vi "UHR-Fleezers Control (host) - 10.5.vi"() -> ()   [LabVIEW 2010] (continued)
        n1065 = local read "Scan Range (V)\n(of steps)"() -> (w2741:dbl)
        n1066 = property on="Scan Range (V)\n(of steps)" class="DigNum (strict)"("Val(Sgnl)"=w2741) -> ()  [unwired: 2 in, 2 out]
      }
    }
    n1067 = node-c288() -> ()  [unwired: 2 out]
  }
  n1068 = node-c288(3 ("Processor")) -> (w77:T25)  [unwired: 3 out]
  n1069 = disable-structure shown="Disabled" {
    disable-tunnel: [w4150 _] -> w13
    disable-tunnel: w9 -> [w4149 _]
    frame Disabled {
      n1070 = node-c288() -> (w4152:T25)  [unwired: 4 out]
      n1071 = timed-loop "Rough control of MCL mirror stage (debugging)" {
        tunnel: w4149 -> [w4155]
        tunnel: [w4154] -> w4150
        timing: w4152 -> [_]
        timing-out: [_] -> w4151
        stop <- w4154 stop-if-true
        n1072 = node-c288() -> ()  [unwired: 2 out]
        n1073 = case shown="1" "MCL Mode" {
          tunnel: w4155 -> [_ w4158 w4262]
          frame 0, Default {
          }
          frame 1 {
            n1074 = node-c288() -> (w4160:T25)  [unwired: 4 out]
            n1075 = timed-loop "Oscillate MCL mirror" {
              timing: w4160 -> [_]
              timing-out: [_] -> w4159
              tunnel: w4158 -> [w4199]
              i -> [w4198]
              stop <- w4161 stop-if-true
              n1076 = node-c288() -> (w4197:i64)  [unwired: 1 out]
              n1077 = Multiply(x="AO1", y=32767.0) -> (x*y=w4193:dbl)
              n1078 = Multiply(x="AO2", y=32767.0) -> (x*y=w4188:dbl)
              n1079 = Divide(x=w4193, y=10.0) -> (x/y=w4194:dbl)
              n1080 = Divide(x=w4188, y=10.0) -> (x/y=w4189:dbl)
              n1081 = To Word Integer(number=w4194) -> (16bit integer=w4186:i16)
              n1082 = To Word Integer(number=w4189) -> (16bit integer=w4185:i16)
              n1083 = Divide(x=w4197, y=i64 1000) -> (x/y=w4168:dbl)
              n1084 = Multiply(x=w4168, y=w4198) -> (x*y=w4179:dbl)
              n1085 = Multiply(x="Osc. freq. (Hz) 2", y=6.283185307179586) -> (x*y=w4180:dbl)
              n1086 = Multiply(x=w4180, y=w4179) -> (x*y=w4178:dbl)
              n1087 = Sine(x=w4178) -> (sin(x)=w4177:dbl)
              n1088 = Multiply(x=w4177, y="Osc. amp. (V)") -> (x*y=w4175:dbl)
              n1089 = Add(x=w4175, y="Osc. center (V)") -> (x+y=w4173:dbl)
              n1090 = Divide(x=w4173, y=10.0) -> (x/y=w4171:dbl)
              n1091 = Multiply(x=w4171, y=32767.0) -> (x*y=w4166:dbl)
              n1092 = Select(t=w4166, s="Scan axis", f=w4186) -> (s? t:f=w4184:dbl)
              n1093 = Select(t=w4185, s="Scan axis", f=w4166) -> (s? t:f=w4183:dbl)
              n1094 = local read "MCL Mode"() -> (w4165:u16)
              n1095 = Not Equal?(x=w4165, y=u16 1) -> (x != y?=w4162:bool)
              n1096 = local read "Stop All"() -> (w4163:bool)
              n1097 = xnode "Read/Write Control"("FPGA VI Reference In"=w4199, "AO1"=w4184, "AO2"=w4183) -> ()  [unwired: 1 in, 2 out]
              n1098 = Compound Arithmetic op=OR(w4163, w4162) -> (w4161:bool)
              n1099 = node-c288() -> ()  [unwired: 2 out]
            }
            n1100 = node-c288(w4159) -> ()  [unwired: 1 out]
          }
          frame 2 {
            n1101 = case shown="True" "Start Scan" {
              tunnel: w4262 -> [_ w4274]
              frame False {
              }
              frame True {
                n1102 = Subtract(x="End (V)", y="Begin (V)") -> (x-y=w4270:dbl)
                n1103 = Decrement(x="N Points") -> (x-1=w4269:dbl)
                n1104 = Divide(x=w4270, y=w4269) -> (x/y=w4267:dbl)
                n1105 = for {
                  N: "N Points" -> [_]
                  tunnel: "Begin (V)" -> [w4287]
                  tunnel: w4274 -> [w4279]
                  tunnel: [w4278] -> w4273 mode=indexing
                  tunnel: w4267 -> [w4277]
                  tunnel: [w4275] -> w4266 mode=indexing
                  i -> [w4286]
                  n1106 = Multiply(x=w4277, y=w4286) -> (x*y=w4285:dbl)
                  n1107 = Add(x=w4287, y=w4285) -> (x+y=w4282:dbl)
                  n1108 = local read "Scan axis"() -> (w4276:bool)
                  n1109 = local read "AO1"() -> (w4284:dbl)
                  n1110 = local read "AO2"() -> (w4283:dbl)
                  n1111 = Select(t=w4282, s=w4276, f=w4284) -> (s? t:f=w4281:dbl)
                  n1112 = Select(t=w4283, s=w4276, f=w4282) -> (s? t:f=w4280:dbl)
                  n1113 = flat-sequence {
                    tunnel: w4281 -> [w4291]
                    tunnel: w4280 -> [w4290]
                    tunnel: w4279 -> [w4288]
                    tunnel: [w4358] -> w4278
                    tunnel: [w4357] -> w4275
                    frame #0 {
                      w4294 = 10.0 ("y")
                      w4289 = 32767.0 ("y")
                      n1114 = Multiply(x=w4291, y=w4289) -> (x*y=w4297:dbl)
                      n1115 = Multiply(x=w4290, y=w4289) -> (x*y=w4295:dbl)
                      n1116 = Divide(x=w4297, y=w4294) -> (x/y=w4298:dbl)
                      n1117 = Divide(x=w4295, y=w4294) -> (x/y=w4296:dbl)
                      n1118 = To Word Integer(number=w4298) -> (16bit integer=w4292:i16)
                      n1119 = To Word Integer(number=w4296) -> (16bit integer=w4293:i16)
                      n1120 = xnode "Read/Write Control"("FPGA VI Reference In"=w4288, "AO1"=w4292, "AO2"=w4293) -> ()  [unwired: 1 in, 2 out]
                    }
                    frame #1 {
                      n1121 = Wait (ms)(milliseconds to wait="DAQ Delay (ms)") -> ()  [unwired: 1 out]
                    }
                    frame #2 {
                      n1122 = local read "Slow mean"() -> (w4358:dbl)
                      n1123 = local read "Sigma"() -> (w4357:dbl)
                    }
                  }
                }
                n1124 = Bundle("Begin (V)"="Begin (V)", w4267, w4273) -> (→"MCL Scan":cluster{"Begin (V)":dbl, dbl, dbl[]})  [unwired: 1 out]
                n1125 = Bundle("Begin (V)"="Begin (V)", w4267, w4266) -> (→"MCL Scan 2":cluster{"Begin (V)":dbl, dbl, dbl[]})  [unwired: 1 out]
              }
            }
          }
        }
        n1126 = local read "Stop All"() -> (w4154:bool)
        n1127 = node-c288() -> ()  [unwired: 2 out]
      }
      n1128 = node-c288(w4151) -> ()  [unwired: 1 out]
    }
    frame Enabled {
    }
  }
  n1129 = timed-loop "Control parameters (event loop)" {
    tunnel: w9 -> [w4365]
    shift-right: [w4364] -> _
    shift-left: errorcluster {"status"=FALSE, "code"=0, "source"=""} ("error out") -> [w4363]
    tunnel: [w4362] -> w15
    timing: w79 -> [_]
    timing-out: [_] -> w78
    tunnel: w56 -> [w4361]
    stop <- w4362 stop-if-true
    n1130 = node-c288() -> ()  [unwired: 2 out]
    n1131 = event shown="[32] Key Down" {
      selector: _ -> [_ _ _ _ _ _ _ _ _ _ _ _ _ _ _ _ _ _ _ _ _ _ _ _ _ _ _ _ _ _ _ _ _ _ _ _ _ _ _ _ _ _ _ _ _ _ _ _ _ _ _ _ _ _]
      dyn-events: _ -> [_ _ _ _ _ _ _ _ _ _ _ _ _ _ _ _ _ _ _ _ _ _ _ _ _ _ _ _ _ _ _ _ _ _ _ _ _ _ _ _ _ _ _ _ _ _ _ _ _ _ _ _ _ _]
      timeout: _ -> [_ _ _ _ _ _ _ _ _ _ _ _ _ _ _ _ _ _ _ _ _ _ _ _ _ _ _ _ _ _ _ _ _ _ _ _ _ _ _ _ _ _ _ _ _ _ _ _ _ _ _ _ _ _]
      tunnel: w4365 -> [w4403 _ _ _ w4525 _ w4622 _ _ _ _ w4688 _ _ w4790 w4934 w4998 w5073 w5227 w5304 w5435 w5531 w5617 w5703 w5789 w5875 w5961 w6054 w6218 w6429 w6572 w6709 _ _ w6955 w6997 w7045 w7124 w7166 _ w7212 _ _ _ _ w7395 _ w7488 w7529 w7576 w7764 w7813 _ w7875]
      tunnel: [w4402 _ _ _ w4515 _ w4621 _ _ w4653 _ w4667 _ _ w4789 w4930 w4995 w5070 w5226 w5302 w5434 w5525 w5611 w5697 w5783 w5869 w5955 w6052 w6217 w6427 w6570 w6707 _ _ w6953 w6995 w7035 w7122 w7164 _ w7210 _ _ _ _ w7393 _ _ _ _ _ _ _ _] -> w4364
      tunnel: w4363 -> [w4401 _ _ _ w4524 _ w4620 _ _ w4653 _ w4687 _ _ w4788 w4929 w4994 w5069 w5225 w5303 w5433 w5530 w5616 w5702 w5788 w5874 w5960 w6053 w6216 w6428 w6571 w6708 _ _ w6954 w6996 w7044 w7123 w7165 _ w7211 _ _ _ _ w7394 _ w7487 w7528 w7575 w7763 w7812 _ w7874]
      tunnel: [_ _ _ _ _ _ _ _ _ w4652 _ _ _ _ _ _ _ _ _ _ _ _ _ _ _ _ _ _ _ _ _ _ _ _ _ _ _ _ _ _ _ _ _ _ _ _ _ _ _ _ _ _ _ _] -> w4362
      tunnel: [_ _ _ _ _ _ _ "Round T1 X" _ _ _ _ _ _ _ _ _ _ _ _ _ _ _ _ _ _ _ _ _ _ _ _ _ _ _ _ _ _ _ _ _ _ _ _ _ _ _ _ _ _ _ _ _ _] -> _
      tunnel: [_ _ _ "Adjust Scale\nto Mean" _ _ _ _ _ _ _ _ _ _ _ _ _ _ _ _ _ _ _ _ _ _ _ _ _ _ _ _ _ _ _ _ _ _ _ _ _ _ _ _ _ _ _ _ _ _ _ "Set SP to Reading" _ _] -> _
      tunnel: [_ _ _ _ _ _ _ _ "Round T2 X" _ "Delayed Interlace Start" _ _ _ _ _ _ _ _ _ _ _ _ _ _ _ _ _ _ _ _ _ _ _ _ _ _ _ _ _ _ _ _ _ _ _ _ _ _ _ _ _ _ _] -> _
      tunnel: w4361 -> [_ _ _ _ _ _ _ _ _ _ _ _ _ _ _ _ _ _ _ _ _ _ _ _ _ _ _ _ _ _ _ _ _ _ _ _ _ _ _ _ _ _ _ _ w7386 _ _ _ _ _ _ _ _ _]
      event "AI Count (ticks)", "Sets to FIFO (Traps)", "Save ave N", "FPGA Ave.", "# Samples/channel", "N sets to save": Value Change {
        # "So that if 'Save ave N' is updated, the AOD scanning code updates too."
        n1132 = event-data() -> ()  [unwired: 6 out]
        n1133 = local read "AI Count (ticks)"() -> (w4383:u32)
        n1134 = Boolean To (0,1)(Boolean="Sets to FIFO (Traps)") -> (0, 1=w4393:cluster{"Set 1":i16, "Set 2":i16, "Set 3":i16})
        n1135 = xnode "Read/Write Control"("FPGA VI Reference In"=w4403, "error in"=w4401, "ai count"=w4383, "AI1 Sets to FIFO"="Sets to FIFO (Traps)", "N of AI1 Int Acq Sets"="N Acq Sets (Traps + Fl.)") -> ("error out"=w4402:errorcluster)  [unwired: 1 out]
        n1136 = Cluster To Array(cluster=w4393) -> (array=w4392:i16[])
        n1137 = To Unsigned Long Integer(number=w4392) -> (unsigned 32bit integer=w4372:u32[])
        n1138 = local read "Scan steps (AOD)"() -> (w4394:u64)
        n1139 = Multiply(x=w4383, y="N Acq Sets (Traps + Fl.)") -> (x*y=w4381:u32)
        n1140 = Divide(x=40000000.0, y=w4383) -> (x/y=w4375:dbl)
        "AI rate (Hz)" <- w4375
        "Ave. Rate (Hz)" <- w4375
        n1141 = Add Array Elements(numeric array=w4372) -> (sum=w4384:u32)
        "Trap Sets" <- w4384
        n1142 = Reciprocal(x=w4375) -> (1/x=→"Ave. Period (s)":dbl)
        n1143 = property on="Scan steps (AOD)" class="DigNum (strict)"("Val(Sgnl)"=w4394) -> ()  [unwired: 2 in, 2 out]
        n1144 = Divide(x=w4375, y="N Acq Sets (Traps + Fl.)") -> (x/y=w4398:dbl)
        "Data Rate (Hz)" <- w4398
        n1145 = Reciprocal(x=w4398) -> (1/x=→"Data Period (s)":dbl)
        n1146 = local read "Save ave N"() -> (w4397:dbl)
        n1147 = Divide(x=w4398, y=w4397) -> (x/y=w4396:dbl)
        "Save Data Rate (Hz)" <- w4396
        n1148 = Reciprocal(x=w4396) -> (1/x=→"Save Data Period (s)":dbl)
        n1149 = Multiply(x=w4381, y="# Samples/trap") -> (x*y=w4379:u32)
        "Counts/DMA" <- w4379
        n1150 = property on="Trap Disp. Downsample" class="DigNum (strict)"("Maximum"="# Samples/trap") -> ()  [unwired: 2 in, 2 out]
        n1151 = Multiply(x=w4384, y="# Samples/trap") -> (x*y=w4373:u32)
        "# Samples/channel" <- w4373
        n1152 = Multiply(x=w4373, y=u32 8) -> (x*y=→"Trap AI Elements/DMA read":u32)
        n1153 = local read "APD Int. Count"() -> (w4380:u32)
        n1154 = Multiply(x=w4373, y=u32 3) -> (x*y=→"Trap Pos Elements/DMA read":u32)
        n1155 = Divide(x=w4379, y=w4380) -> (x/y=w4370:dbl)
        "APD Samples/FIFO Acq." <- w4370
        n1156 = Divide(x=w4379, y=40000000.0) -> (x/y=w4377:dbl)
        "DMA Update Period (s)" <- w4377
        n1157 = Multiply(x=2.0, y=w4370) -> (x*y=→"APD Elements/DMA read":dbl)
        n1158 = property on="APD Disp. Downsample" class="DigNum (strict)"("Maximum"=w4370) -> ()  [unwired: 2 in, 2 out]
        n1159 = local read "N sets to save"() -> (w4390:u32)
        n1160 = Multiply(x=w4377, y=w4390) -> (x*y=→"Total Time (s)":dbl)
        "FPGA Averaging" <- FALSE ("FPGA Averaging")
      }
      event "Rescale on Mean": Value Change {
        n1161 = event-data() -> ()  [unwired: 7 out]
        n1162 = And(x=FALSE, y="Rescale on Mean") -> (x .and. y?=w4490:bool)
        n1163 = local write "Rescale on Mean"(w4490) -> ()
        n1164 = local read "Bead Mean (nm)"() -> (w4495:dbl)
        n1165 = Add(x="Amplitude (nm)", y=w4495) -> (x+y=w4493:dbl)
        n1166 = Subtract(x=w4495, y="Amplitude (nm)") -> (x-y=w4492:dbl)
        n1167 = property on="Bead Separation" class="WFChart (strict)"("YScale.Minimum"=w4492) -> ()  [unwired: 2 in, 2 out]
        n1168 = property on="Bead Separation" class="WFChart (strict)"("YScale.Maximum"=w4493) -> ()  [unwired: 2 in, 2 out]
      }
      event "Detector Type": Value Change {
        n1169 = event-data() -> ()  [unwired: 7 out]
        n1170 = local read "AI labels"() -> (w4496:string[])
        n1171 = property on="High Res. Display" class="Ring (strict)"("Strings []"=w4496) -> ()  [unwired: 2 in, 2 out]
        n1172 = Build Array (concatenate)(w4496, "none") -> (w4497:string[])
        n1173 = property on="FFT 1 Choice 1" class="Ring (strict)"("Strings []"=w4497) -> ()  [unwired: 2 in, 2 out]
        n1174 = property on="FFT 1 Choice 2" class="Ring (strict)"("Strings []"=w4497) -> ()  [unwired: 2 in, 2 out]
        n1175 = property on="FFT 2 Choice 1" class="Ring (strict)"("Strings []"=w4497) -> ()  [unwired: 2 in, 2 out]
        n1176 = property on="FFT 2 Choice 2" class="Ring (strict)"("Strings []"=w4497) -> ()  [unwired: 2 in, 2 out]
        n1177 = Bundle("APD 1", "APD 2") -> (w4500:cluster{string, string})  [unwired: 1 out]
        n1178 = Cluster To Array(cluster=w4500) -> (array=w4498:string[])
        n1179 = Build Array (concatenate)(w4498, w4497) -> (w4502:string[])
        n1180 = Array Size(array=w4502) -> (size(s)=w4503:i32)
        n1181 = property on="Signals to Plot" class="LstBox (strict)"("Item Names"=w4502) -> ()  [unwired: 2 in, 2 out]
        n1182 = property on="Signals to Plot" class="LstBox (strict)"("Number of Rows"=w4503) -> ()  [unwired: 2 in, 2 out]
        n1183 = property on="All Signals" class="WFChart (strict)"("LegNumRows"=w4503) -> ()  [unwired: 2 in, 2 out]
      }
      event "Adjust Scale\nto Mean": Value Change {
        n1184 = event-data() -> ()  [unwired: 7 out]
        n1185 = local read "APD 1 Rate (Hz)"() -> (w4512:dbl)
        n1186 = Multiply(x=1000.0, y="Above (kHz)") -> (x*y=w4510:dbl)
        n1187 = Multiply(x=1000.0, y="Below (kHz)") -> (x*y=w4508:dbl)
        n1188 = Add(x=w4510, y=w4512) -> (x+y=w4505:dbl)
        n1189 = Subtract(x=w4512, y=w4508) -> (x-y=w4506:dbl)
        n1190 = property on="APD Chart" class="WFChart (strict)"("YScale.Minimum"=w4506) -> ()  [unwired: 2 in, 2 out]
        n1191 = property on="APD Chart" class="WFChart (strict)"("YScale.Maximum"=w4505) -> ()  [unwired: 2 in, 2 out]
      }
      event "Phase adj. (AI1)", "+ phase (AI1)", "- phase (AI1)": Value Change {
        n1192 = event-data() -> ()  [unwired: 7 out]
        n1193 = Negate(x="Phase adj. (AI1)") -> (-x=w4522:i16)
        n1194 = Select(t=w4522, s="- phase (AI1)", f="Phase adj. (AI1)") -> (s? t:f=w4521:i16)
        n1195 = xnode "Read/Write Control"("FPGA VI Reference In"=w4525, "error in"=w4524, "Phase count adjustment"=w4521) -> ("FPGA VI Reference Out"=w4520:T20, "error out"=w4519:errorcluster)
        n1196 = Or(x="- phase (AI1)", y="+ phase (AI1)") -> (x .or. y?=w4516:bool)
        n1197 = xnode "Read/Write Control"("FPGA VI Reference In"=w4520, "error in"=w4519, "+ phase"=w4516) -> ("error out"=w4515:errorcluster)  [unwired: 1 out]
      }
      event "Signals to Plot": Double Click {
        w4603 = u32 9868950 ("Color Box")
        n1198 = event-data() -> ("Row"=w4605:i32)  [unwired: 9 out]
        n1199 = property on="All Signals" class="WFChart (strict)"("Active Plot"=w4605) -> (error out=w4616:errorcluster)  [unwired: 2 in, 1 out]
        n1200 = property on="All Signals" class="WFChart (strict)" props=["Plot", "Visible?", "Plot", "Plot Color"](error in=w4616) -> (error out=w4615:errorcluster, "Plot.Visible?"=w4614:bool)  [unwired: 1 in, 2 out]
        n1201 = Select(t=FALSE ("Plot.Visible"), s=w4614, f=TRUE ("Plot.Visible")) -> (s? t:f=w4609:bool)
        n1202 = property on="All Signals" class="WFChart (strict)"(error in=w4615, "Plot.Visible?"=w4609) -> (error out=w4611:errorcluster)  [unwired: 1 in, 1 out]
        n1203 = property on="All Signals" class="WFChart (strict)"(error in=w4611) -> (error out=w4606:errorcluster, "Plot.Plot Color"=w4610:u32)  [unwired: 1 in, 1 out]
        n1204 = property on="Signals to Plot" class="LstBox (strict)"(error in=w4606, "Active Row"=w4605) -> (error out=w4604:errorcluster)  [unwired: 1 in, 1 out]
        n1205 = Select(t=w4610, s=w4609, f=u32 0) -> (s? t:f=w4607:u32)
        n1206 = property on="Signals to Plot" class="LstBox (strict)"(error in=w4604, "CellFontColor"=w4607, "SelColor"=w4603, "CellBG"=w4603, "CellFontSize"=u32 20 ("Active Row:Cell Font:Size"), "CellFontBold"=TRUE ("Active Row:Cell Font:Bold")) -> ()  [unwired: 1 in, 2 out]
      }
      event "BD 1 Frequency 1 (MHz)", "BD 1 Frequency 2 (MHz)", "BD 1 Frequency 3 (MHz)", "BD 2 Frequency 1 (MHz)", "BD 2 Frequency 2 (MHz)", "BD 2 Frequency 3 (MHz)", "Trap Delta (MHz)": Value Change {
        # "anytime one of the frequencies is changed, write it to the RF board UNLESS Set 1 is being oscillated. The oscillation\nscript writes the frequencies to the RF board."
        n1207 = event-data() -> ("CtlRef"=w4619:refnum<vi>)  [unwired: 6 out]
        n1208 = control-ref of="Trap Delta (MHz)"() -> (w4618:refnum<vi>)
        n1209 = Equal?(x=w4618, y=w4619) -> (x = y?=w4617:bool)
        n1210 = case shown="False" "Oscillate Set 1" {
          tunnel: w4622 -> [w4642 _]
          tunnel: [w4641 w4645] -> w4621
          tunnel: w4620 -> [w4640 w4645]
          tunnel: w4617 -> [w4625 _]
          frame False {
            n1211 = local read "BD 1 Frequency 2 (MHz)"() -> (w4629:dbl)
            n1212 = local read "BD 1 Frequency 1 (MHz)"() -> (w4627:dbl)
            n1213 = Subtract(x=w4629, y="Trap Delta (MHz)") -> (x-y=w4626:dbl)
            n1214 = Select(t=w4626, s=w4625, f=w4627) -> (s? t:f=w4624:dbl)
            n1215 = local read "Y RF Frequency Limits (MHz)"() -> (w4630:T17)
            n1216 = local read "X RF Frequency Limits (MHz)"() -> (w4631:T17)
            n1217 = local read "BD 1 Frequency 3 (MHz)"() -> (w4643:dbl)
            n1218 = local write "BD 1 Frequency 1 (MHz)"(w4624) -> ()
            n1219 = local read "BD 2 Frequency 1 (MHz)"() -> (w4634:dbl)
            n1220 = local read "BD 2 Frequency 2 (MHz)"() -> (w4633:dbl)
            n1221 = local read "BD 2 Frequency 3 (MHz)"() -> (w4644:dbl)
            n1222 = call "set RF board frequency - interlace.vi"("Board 2 Frequency Limits"=w4630, "Board 1 Frequency Limits"=w4631, "error in"=w4640, "FPGA VI Reference In"=w4642, "Board 2 Frequency 3 (MHz)"=w4644, "Board 1 Frequency 3 (MHz)"=w4643, "Board 2 Frequency 2 (MHz)"=w4633, "Board 2 Frequency 1 (MHz)"=w4634, "Board 1 Frequency 2 (MHz)"=w4629, "Board 1 Frequency 1  (MHz)"=w4624) -> ("error out"=w4641:errorcluster)  [unwired: 1 out]
            n1223 = Subtract(x=w4634, y=w4633) -> (x-y=w4638:dbl)
            n1224 = Subtract(x=w4624, y=w4629) -> (x-y=w4639:dbl)
            n1225 = Square(x=w4638) -> (x^2=w4636:dbl)
            n1226 = Square(x=w4639) -> (x^2=w4637:dbl)
            n1227 = Add(x=w4637, y=w4636) -> (x+y=w4635:dbl)
            n1228 = Square Root(x=w4635) -> (sqrt(x)=w4632:dbl)
            n1229 = local write "Trap Delta (MHz)"(w4632) -> ()
            n1230 = property on="Initial delta (MHz)" class="DigNum (strict)"("Val(Sgnl)"=w4632) -> ()  [unwired: 2 in, 2 out]
          }
          frame True {
          }
        }
      }
      event "Round T1 X": Value Change {
        n1231 = event-data() -> ()  [unwired: 7 out]
        n1232 = local read "BD 1 Frequency 1 (MHz)"() -> (w4648:dbl)
        n1233 = Round To Nearest(number=w4648) -> (nearest integer value=w4647:dbl)
        n1234 = property on="BD 1 Frequency 1 (MHz)" class="DigNum (strict)"("Val(Sgnl)"=w4647) -> ()  [unwired: 2 in, 2 out]
      }
      event "Round T2 X": Value Change {
        n1235 = event-data() -> ()  [unwired: 7 out]
        n1236 = local read "BD 1 Frequency 2 (MHz)"() -> (w4650:dbl)
        n1237 = Round To Nearest(number=w4650) -> (nearest integer value=w4649:dbl)
        n1238 = property on="BD 1 Frequency 2 (MHz)" class="DigNum (strict)"("Val(Sgnl)"=w4649) -> ()  [unwired: 2 in, 2 out]
      }
      event "Stop All": Value Change {
        n1239 = event-data() -> ()  [unwired: 7 out]
        n1240 = local read "Stop All"() -> (w4652:bool)
      }
      event "Delayed Interlace Start": Value Change {
        n1241 = event-data() -> ()  [unwired: 7 out]
        n1242 = flat-sequence {
          frame #0 {
            n1243 = Multiply(x="Delay to Interlace (s)", y=1000.0) -> (x*y=w4655:dbl)
            n1244 = Wait (ms)(milliseconds to wait=w4655) -> ()  [unwired: 1 out]
          }
          frame #1 {
            n1245 = property on="Green laser mode" class="RadioBtnsControl (strict)"("Val(Sgnl)"=enum32{"Laser ON", "Laser OFF", "Interlace"}."Interlace" ("Value (Signaling)")) -> ()  [unwired: 2 in, 2 out]
          }
        }
      }
      event "BD 1 Amplitude 1 (%)", "BD 1 Amplitude 2 (%)", "BD 1 Amplitude 3 (%)", "BD 2 Amplitude 1 (%)", "BD 2 Amplitude 2 (%)", "BD 2 Amplitude 3 (%)", "Trap 1 ON", "Trap 2 ON", "Trap 3 ON", "Feedback On/Off", "All FB On/Off": Value Change {
        w4679 = i16 1 ("f")
        n1246 = event-data() -> ()  [unwired: 7 out]
        n1247 = local write "Trap 1 (ON/OFF)"("Trap 1 ON") -> ()
        n1248 = local write "Trap 2 (ON/OFF)"("Trap 2 ON") -> ()
        n1249 = Boolean To (0,1)(Boolean="Trap 3 ON") -> (0, 1=w4680:i16)
        n1250 = Boolean To (0,1)(Boolean="Trap 1 ON") -> (0, 1=w4681:i16)
        n1251 = Boolean To (0,1)(Boolean="Trap 2 ON") -> (0, 1=w4682:i16)
        n1252 = Select(t=w4682, s="Trap ON/OFF X or Y Amp?", f=w4679) -> (s? t:f=w4677:i16)
        n1253 = Select(t=w4681, s="Trap ON/OFF X or Y Amp?", f=w4679) -> (s? t:f=w4678:i16)
        n1254 = Select(t=w4680, s="Trap ON/OFF X or Y Amp?", f=w4679) -> (s? t:f=w4676:i16)
        n1255 = Select(t=w4679, s="Trap ON/OFF X or Y Amp?", f=w4682) -> (s? t:f=w4674:i16)
        n1256 = Select(t=w4679, s="Trap ON/OFF X or Y Amp?", f=w4681) -> (s? t:f=w4675:i16)
        n1257 = Select(t=w4679, s="Trap ON/OFF X or Y Amp?", f=w4680) -> (s? t:f=w4673:i16)
        n1258 = And(x="All FB On/Off", y="Feedback On/Off") -> (x .and. y?=w4671:cluster{"Set 1":bool, "Set 2":bool})
        n1259 = local read "BD 1 Amplitude 1 (%)"() -> (w4691:dbl)
        n1260 = local read "BD 1 Amplitude 2 (%)"() -> (w4690:dbl)
        n1261 = local read "BD 1 Amplitude 3 (%)"() -> (w4689:dbl)
        n1262 = Unbundle By Name(w4671) -> ("Set 1"=w4666:bool, "Set 2"=w4663:bool)
        n1263 = local read "Y RF Amplitude Limits (%)"() -> (w4659:T17)
        n1264 = local read "X RF Amplitude Limits (%)"() -> (w4660:T17)
        n1265 = local read "BD 2 Amplitude 1 (%)"() -> (w4692:dbl)
        n1266 = local read "BD 2 Amplitude 2 (%)"() -> (w4693:dbl)
        n1267 = local read "BD 2 Amplitude 3 (%)"() -> (w4694:dbl)
        n1268 = And(x="Trap 2 ON", y=w4663) -> (x .and. y?=w4661:bool)
        n1269 = And(x="Trap 1 ON", y=w4666) -> (x .and. y?=w4664:bool)
        n1270 = Multiply(x=w4678, y=w4691) -> (x*y=w4686:dbl)
        n1271 = Multiply(x=w4690, y=w4677) -> (x*y=w4684:dbl)
        n1272 = Multiply(x=w4689, y=w4676) -> (x*y=w4685:dbl)
        n1273 = Multiply(x=w4692, y=w4675) -> (x*y=w4695:dbl)
        n1274 = Multiply(x=w4693, y=w4674) -> (x*y=w4696:dbl)
        n1275 = Multiply(x=w4694, y=w4673) -> (x*y=w4697:dbl)
        n1276 = call "set RF board amplitude - interlace.vi"("Board 2 Amplitude Limits"=w4659, "Board 1 Amplitude Limits"=w4660, "error in"=w4687, "FPGA VI Reference In"=w4688, "Board 2 Amplitude 3 (%)"=w4697, "Board 1 Amplitude 3 (%)"=w4685, "Board 2 Amplitude 2 (%)"=w4696, "Board 2 Amplitude 1 (%)"=w4695, "Board 1 Amplitude 2 (%)"=w4684, "Board 1 Amplitude 1 (%)"=w4686) -> ("error out"=w4668:errorcluster, "FPGA VI Reference Out"=w4669:T20)
        n1277 = xnode "Read/Write Control"("FPGA VI Reference In"=w4669, "error in"=w4668, "FB On/Off Set 1"=w4664, "FB On/Off Set 2"=w4661) -> ("error out"=w4667:errorcluster)  [unwired: 1 out]
      }
      event "Load parameters": Value Change {
        n1278 = event-data() -> ()  [unwired: 7 out]
        n1279 = property on="Saved AOD Raster Scan Parameter Sets" class="Arr (strict)"() -> ("Index Values"=w4767:u32[])  [unwired: 2 in, 2 out]
        n1280 = Index Array(array=w4767, index=0) -> (element=w4764:u32)
        n1281 = local write "Load parameters"(FALSE ("Load parameters")) -> ()
        n1282 = Index Array(array="Saved AOD Raster Scan Parameter Sets", index=w4764) -> (element=w4763:T46)
        n1283 = Unbundle By Name(w4763) -> ("Scan Range AOD (nm) 2"=w4762:dbl, "Step Size AOD (nm) 2"=w4761:dbl, "Scan Speed AOD (nm/s) 2"=w4760:dbl, "Number of scans (AOD) 2"=w4759:u16)
        n1284 = flat-sequence {
          tunnel: w4762 -> [w4770]
          tunnel: w4761 -> [w4769]
          tunnel: w4760 -> [w4768]
          tunnel: w4759 -> [w4771]
          frame #0 {
            n1285 = local write "Scan Speed (nm/s)"(w4768) -> ()
            n1286 = local write "Scan Range (nm)"(w4770) -> ()
            n1287 = local write "Step Size (nm)"(w4769) -> ()
          }
          frame #1 {
            n1288 = property on="Number of F/B Scans (AOD)" class="DigNum (strict)"("Val(Sgnl)"=w4771) -> ()  [unwired: 2 in, 2 out]
          }
        }
      }
      event "Trap 1 (ON/OFF)", "Trap 2 (ON/OFF)": Value Change {
        n1289 = event-data() -> ()  [unwired: 7 out]
        n1290 = property on="Trap 2 ON" class="Bool (strict)"("Val(Sgnl)"="Trap 2 (ON/OFF)") -> ()  [unwired: 2 in, 2 out]
        n1291 = property on="Trap 1 ON" class="Bool (strict)"("Val(Sgnl)"="Trap 1 (ON/OFF)") -> ()  [unwired: 2 in, 2 out]
      }
      event "DIO count 1 (ticks)", "DIO count 2 (ticks)", "DIO count 3 (ticks)", "Interlace", "Number Interlace Sets", "Not-Interlacing Set": Value Change {
        n1292 = event-data() -> ()  [unwired: 7 out]
        n1293 = local read "DIO count 3 (ticks)"() -> (w4784:u32)
        n1294 = local read "DIO count 1 (ticks)"() -> (w4786:u32)
        n1295 = local read "DIO count 2 (ticks)"() -> (w4785:u32)
        n1296 = To Unsigned Byte Integer(number="Not-Interlacing Set") -> (unsigned 8bit integer=w4775:u8)
        n1297 = Add(x=w4775, y=u8 1) -> (x+y=w4779:u8)
        n1298 = xnode "Read/Write Control"("FPGA VI Reference In"=w4790, "error in"=w4788, "DIO count 1 (ticks)"=w4786, "DIO count 2 (ticks)"=w4785, "DIO count 3 (ticks)"=w4784, "Interlace ON/OFF"="Interlace", "Number Interlace Cycles"="Number Interlace Sets", "Interlace Off Parameters"=w4779) -> ("error out"=w4789:errorcluster)  [unwired: 1 out]
        n1299 = Build Array(w4786, w4785, w4784) -> (w4777:u32[])
        n1300 = Split 1D Array(array=w4777, index="Number Interlace Sets") -> (first subarray=w4787:u32[])  [unwired: 1 out]
        n1301 = Index Array(array=w4777, index=w4775) -> (element=w4776:u32)
        n1302 = Add Array Elements(numeric array=w4787) -> (sum=w4781:u32)
        n1303 = Select(t=w4781, s="Interlace", f=w4776) -> (s? t:f=→"Total Counts (ticks)":u32)
      }
      event "Reset Feedback": Value Change {
        n1304 = event-data() -> ()  [unwired: 7 out]
        n1305 = Unbundle By Name("Reset Feedback") -> ("Set 1"=w4932:bool, "Set 2"=w4931:bool)
        n1306 = xnode "Read/Write Control"("FPGA VI Reference In"=w4934, "error in"=w4929, "FB Reset Set 1"=w4932, "FB Reset Set 2"=w4931) -> ("error out"=w4930:errorcluster)  [unwired: 1 out]
      }
      event "PID Gains": Value Change {
        n1307 = event-data() -> ()  [unwired: 7 out]
        n1308 = Unbundle By Name("PID Gains") -> ("Set 1"=w4997:T15, "Set 2"=w4996:T15)
        n1309 = xnode "Read/Write Control"("FPGA VI Reference In"=w4998, "error in"=w4994, "FB Gains Set 1"=w4997, "FB Gains Set 2"=w4996) -> ("error out"=w4995:errorcluster)  [unwired: 1 out]
      }
      event "AI2 to Setpoint", "Trap Intensity\nSetpoints (V)": Value Change {
        n1310 = event-data() -> ()  [unwired: 7 out]
        n1311 = xnode "Read/Write Control"("FPGA VI Reference In"=w5073, "error in"=w5069) -> ("FPGA VI Reference Out"=w5072:T20, "error out"=w5071:errorcluster, "AI2 Y Sum Set 1"=w5080:i16, "AI2 Y Sum Set 2"=w5079:i16)
        n1312 = Cluster To Array(cluster="AI2 to Setpoint") -> (array=w5083:bool[])
        n1313 = local read "AI2 (V)"() -> (w5081:cluster{"Set 1":dbl, "Set 2":dbl})
        n1314 = Or Array Elements(Boolean array=w5083) -> (logical OR=w5084:bool)
        n1315 = Bundle By Name(cluster=w5081, "Set 1"=w5080, "Set 2"=w5079) -> (w5078:cluster{"Set 1":dbl, "Set 2":dbl})
        n1316 = Divide(x=w5078, y=3276.7) -> (x/y=w5077:cluster{"Set 1":dbl, "Set 2":dbl})
        "AI2 (V)" <- w5077
        n1317 = case shown="True" w5084 {
          tunnel: [w5148 w5165] -> w5076
          tunnel: "AI2 to Setpoint" -> [_ w5161]
          tunnel: "Trap Intensity\nSetpoints (V)" -> [w5149 w5164]
          tunnel: w5077 -> [_ w5158]
          frame False {
            n1318 = Multiply(x=3276.7, y=w5149) -> (x*y=w5150:cluster{"Set 1":dbl, "Set 2":dbl})
            n1319 = To Word Integer(number=w5150) -> (16bit integer=w5148:cluster{"Set 1":i16, "Set 2":i16})
          }
          frame True {
            n1320 = Unbundle By Name(w5158) -> ("Set 1"=w5157:dbl, "Set 2"=w5156:dbl)
            n1321 = Unbundle By Name(w5164) -> ("Set 1"=w5163:dbl, "Set 2"=w5162:dbl)
            n1322 = Unbundle By Name(w5161) -> ("Set 1"=w5160:bool, "Set 2"=w5159:bool)
            n1323 = Select(t=w5157, s=w5160, f=w5163) -> (s? t:f=w5155:dbl)
            n1324 = Select(t=w5156, s=w5159, f=w5162) -> (s? t:f=w5154:dbl)
            n1325 = Bundle By Name(cluster=w5164, "Set 1"=w5155, "Set 2"=w5154) -> (w5152:cluster{"Set 1":dbl, "Set 2":dbl})
            n1326 = local write "Trap Intensity\nSetpoints (V)"(w5152) -> ()
            n1327 = Multiply(x=3276.7, y=w5152) -> (x*y=w5153:cluster{"Set 1":dbl, "Set 2":dbl})
            n1328 = To Word Integer(number=w5153) -> (16bit integer=w5165:cluster{"Set 1":i16, "Set 2":i16})
          }
        }
        n1329 = Unbundle By Name(w5076) -> ("Set 1"=w5075:i16, "Set 2"=w5074:i16)
        n1330 = xnode "Read/Write Control"("FPGA VI Reference In"=w5072, "error in"=w5071, "FB Setpoint Set 1"=w5075, "FB Setpoint Set 2"=w5074) -> ("error out"=w5070:errorcluster)  [unwired: 1 out]
      }
      event "Invert GI": Value Change {
        n1331 = event-data() -> ()  [unwired: 7 out]
        n1332 = xnode "Read/Write Control"("FPGA VI Reference In"=w5227, "error in"=w5225, "Invert GI"="Invert GI", "Invert GI 2"="Invert GI") -> ("error out"=w5226:errorcluster)  [unwired: 1 out]
      }
      event "Green FB Setpoint (mV)", "Green FB Gains", "Green FB On/Off", "Current When FB OFF (%)", "Green int current ON count adj": Value Change {
        n1333 = event-data() -> ()  [unwired: 7 out]
        n1334 = local read "Green FB Setpoint (mV)"() -> (w5293:dbl)
        n1335 = local read "Current When FB OFF (%)"() -> (w5296:dbl)
        n1336 = Multiply(x=w5293, y=3.2767) -> (x*y=w5292:dbl)
        n1337 = Multiply(x=w5296, y=655.35) -> (x*y=w5297:dbl)
        n1338 = To Unsigned Word Integer(number=w5297) -> (unsigned 16bit integer=w5295:u16)
        n1339 = local read "Green int current ON count adj"() -> (w5300:u32)
        n1340 = local read "Green FB Gains"() -> (w5299:T15)
        n1341 = local read "Green Laser ON/Interlacing"() -> (w5290:bool)
        n1342 = local read "Green laser mode"() -> (w5289:enum32{"Laser ON", "Laser OFF", "Interlace"})
        n1343 = local read "Green FB On/Off"() -> (w5301:bool)
        n1344 = Equal?(x=w5289, y=enum32{"Laser ON", "Laser OFF", "Interlace"}."Interlace") -> (x = y?=w5287:bool)
        n1345 = Compound Arithmetic op=AND(w5287, w5301, w5290) -> (w5291:bool)
        n1346 = xnode "Read/Write Control"("FPGA VI Reference In"=w5304, "error in"=w5303, "Green FB Setpoint"=w5292, "Green FB On/Off"=w5291, "Current Out"=w5295, "Green int current ON count adj"=w5300, "Green FB Gains"=w5299) -> ("error out"=w5302:errorcluster)  [unwired: 1 out]
      }
      event "Green laser mode", "Green Laser ON/Interlacing": Value Change {
        n1347 = event-data() -> ()  [unwired: 7 out]
        n1348 = case shown="True" "Green Laser ON/Interlacing" {
          tunnel: "Green laser mode" -> [_ w5442]
          tunnel: [enum32{"Laser ON", "Laser OFF", "Interlace"}."Laser OFF" ("Green laser mode") w5442] -> w5430
          tunnel: [FALSE w5438] -> w5429
          frame False {
          }
          frame True {
            n1349 = local read "Green FB On/Off"() -> (w5439:bool)
            n1350 = Equal?(x=w5442, y=enum32{"Laser ON", "Laser OFF", "Interlace"}."Interlace") -> (x = y?=w5440:bool)
            n1351 = And(x=w5440, y=w5439) -> (x .and. y?=w5438:bool)
          }
        }
        n1352 = xnode "Read/Write Control"("FPGA VI Reference In"=w5435, "error in"=w5433, "Operating Mode"=w5430, "Operating Mode 2"=w5430, "Green FB On/Off"=w5429) -> ("error out"=w5434:errorcluster)  [unwired: 1 out]
      }
      event "- phase (APD 1 Gate)", "+ phase (APD 1 Gate)": Value Change {
        n1353 = event-data() -> ()  [unwired: 7 out]
        n1354 = local read "Phase Adj. (APD 1 Gate)"() -> (w5521:i16)
        n1355 = Negate(x=w5521) -> (-x=w5529:i16)
        n1356 = Select(t=w5529, s="- phase (APD 1 Gate)", f=w5521) -> (s? t:f=w5528:i16)
        n1357 = Or(x="- phase (APD 1 Gate)", y="+ phase (APD 1 Gate)") -> (x .or. y?=w5524:bool)
        n1358 = xnode "Read/Write Control"("FPGA VI Reference In"=w5531, "error in"=w5530, "Phase count adjustment (APD 1 Gate)"=w5528) -> ("FPGA VI Reference Out"=w5526:T20, "error out"=w5527:errorcluster)
        n1359 = xnode "Read/Write Control"("FPGA VI Reference In"=w5526, "error in"=w5527, "+ phase (APD 1 Gate)"=w5524) -> ("error out"=w5525:errorcluster)  [unwired: 1 out]
      }
      event "+ phase (APD 2 Gate)", "- phase (APD 2 Gate)": Value Change {
        n1360 = event-data() -> ()  [unwired: 7 out]
        n1361 = local read "Phase Adj. (APD 2 Gate)"() -> (w5607:i16)
        n1362 = Negate(x=w5607) -> (-x=w5615:i16)
        n1363 = Select(t=w5615, s="- phase (APD 2 Gate)", f=w5607) -> (s? t:f=w5614:i16)
        n1364 = Or(x="- phase (APD 2 Gate)", y="+ phase (APD 2 Gate)") -> (x .or. y?=w5610:bool)
        n1365 = xnode "Read/Write Control"("FPGA VI Reference In"=w5617, "error in"=w5616, "Phase count adjustment (APD 2 Gate)"=w5614) -> ("FPGA VI Reference Out"=w5612:T20, "error out"=w5613:errorcluster)
        n1366 = xnode "Read/Write Control"("FPGA VI Reference In"=w5612, "error in"=w5613, "+ phase (APD 2 Gate)"=w5610) -> ("error out"=w5611:errorcluster)  [unwired: 1 out]
      }
      event "Phase Adj. (APD Acq)", "+ phase (APD Acq)", "- phase (APD Acq)": Value Change {
        n1367 = event-data() -> ()  [unwired: 7 out]
        n1368 = local read "Phase Adj. (APD Acq)"() -> (w5695:i16)
        n1369 = Negate(x=w5695) -> (-x=w5701:i16)
        n1370 = Select(t=w5701, s="+ phase (APD Acq)", f=w5695) -> (s? t:f=w5700:i16)
        n1371 = Or(x="+ phase (APD Acq)", y="- phase (APD Acq)") -> (x .or. y?=w5696:bool)
        n1372 = xnode "Read/Write Control"("FPGA VI Reference In"=w5703, "error in"=w5702, "Phase Count Adjustment (APD Acq)"=w5700) -> ("FPGA VI Reference Out"=w5698:T20, "error out"=w5699:errorcluster)
        n1373 = xnode "Read/Write Control"("FPGA VI Reference In"=w5698, "error in"=w5699, "+ phase (APD Acq)"=w5696) -> ("error out"=w5697:errorcluster)  [unwired: 1 out]
      }
      event "Phase adj. (GI)", "+ phase (GI)", "- phase (GI)": Value Change {
        n1374 = event-data() -> ()  [unwired: 7 out]
        n1375 = Negate(x="Phase adj. (GI)") -> (-x=w5787:i16)
        n1376 = Select(t=w5787, s="+ phase (GI)", f="Phase adj. (GI)") -> (s? t:f=w5786:i16)
        n1377 = Or(x="+ phase (GI)", y="- phase (GI)") -> (x .or. y?=w5782:bool)
        n1378 = xnode "Read/Write Control"("FPGA VI Reference In"=w5789, "error in"=w5788, "Phase count adjustment (GI)"=w5786) -> ("FPGA VI Reference Out"=w5784:T20, "error out"=w5785:errorcluster)
        n1379 = xnode "Read/Write Control"("FPGA VI Reference In"=w5784, "error in"=w5785, "+ phase (GI)"=w5782) -> ("error out"=w5783:errorcluster)  [unwired: 1 out]
      }
      event "Phase adj. (GI) 2", "+ phase (GI) 2", "- phase (GI) 2": Value Change {
        n1380 = event-data() -> ()  [unwired: 7 out]
        n1381 = Negate(x="Phase adj. (GI) 2") -> (-x=w5873:i16)
        n1382 = Select(t=w5873, s="+ phase (GI) 2", f="Phase adj. (GI) 2") -> (s? t:f=w5872:i16)
        n1383 = Or(x="+ phase (GI) 2", y="- phase (GI) 2") -> (x .or. y?=w5868:bool)
        n1384 = xnode "Read/Write Control"("FPGA VI Reference In"=w5875, "error in"=w5874, "Phase count adjustment (GI) 2"=w5872) -> ("FPGA VI Reference Out"=w5870:T20, "error out"=w5871:errorcluster)
        n1385 = xnode "Read/Write Control"("FPGA VI Reference In"=w5870, "error in"=w5871, "+ phase (GI) 2"=w5868) -> ("error out"=w5869:errorcluster)  [unwired: 1 out]
      }
      event "Phase adj. (Green FB)", "- phase (Green FB)", "+ phase (Green FB)": Value Change {
        n1386 = event-data() -> ()  [unwired: 7 out]
        n1387 = Negate(x="Phase adj. (Green FB)") -> (-x=w5959:i16)
        n1388 = Select(t=w5959, s="+ phase (Green FB)", f="Phase adj. (Green FB)") -> (s? t:f=w5958:i16)
        n1389 = Or(x="+ phase (Green FB)", y="- phase (Green FB)") -> (x .or. y?=w5954:bool)
        n1390 = xnode "Read/Write Control"("FPGA VI Reference In"=w5961, "error in"=w5960, "Phase count adjustment (Green FB)"=w5958) -> ("FPGA VI Reference Out"=w5956:T20, "error out"=w5957:errorcluster)
        n1391 = xnode "Read/Write Control"("FPGA VI Reference In"=w5956, "error in"=w5957, "+ phase (Green FB)"=w5954) -> ("error out"=w5955:errorcluster)  [unwired: 1 out]
      }
      event "Invert APD Gate", "APD Gate ON Count", "APD Gate OFF Count", "APD Gate", "APD Integration Time (s)", "APD 1 AO Mult.", "APD 2 AO Mult.": Value Change {
        n1392 = event-data() -> ()  [unwired: 7 out]
        n1393 = local read "APD Integration Time (s)"() -> (w6037:dbl)
        n1394 = local read "APD Gate ON Count"() -> (w6050:u32)
        n1395 = local read "APD Gate OFF Count"() -> (w6049:u32)
        n1396 = local read "Invert APD Gate"() -> (w6051:bool)
        n1397 = local read "APD Gate"() -> (w6048:enum32{"ON", "OFF", "Interlace"})
        n1398 = Multiply(x=w6037, y=40000000.0) -> (x*y=w6046:dbl)
        n1399 = Reciprocal(x=w6037) -> (1/x=→"APD Acq Rate (Hz)":dbl)
        n1400 = To Unsigned Long Integer(number=w6046) -> (unsigned 32bit integer=w6045:u32)
        n1401 = local read "DMA Update Period (s)"() -> (w6038:dbl)
        n1402 = Divide(x=w6038, y=w6037) -> (x/y=w6041:dbl)
        n1403 = local read "APD 1 AO Mult."() -> (w6043:i16)
        n1404 = local read "APD 2 AO Mult."() -> (w6042:i16)
        n1405 = Multiply(x=2.0, y=w6041) -> (x*y=w6040:dbl)
        n1406 = local write "APD Samples/FIFO Acq."(w6041) -> ()
        n1407 = local write "APD Elements/DMA read"(w6040) -> ()
        n1408 = xnode "Read/Write Control"("FPGA VI Reference In"=w6054, "error in"=w6053, "Invert APD Gate"=w6051, "APD Gate ON Count"=w6050, "APD Gate OFF Count"=w6049, "APD Acq Rate Count"=w6045, "APD Gate Operating Mode"=w6048, "APD 1 AO scale factor"=w6043, "APD 2 AO scale factor"=w6042) -> ("error out"=w6052:errorcluster)  [unwired: 1 out]
      }
      event "GI Frequency, ON count", "Green FB Count", "GI Frequency, OFF count": Value Change {
        n1409 = event-data() -> ()  [unwired: 7 out]
        n1410 = xnode "Read/Write Control"("FPGA VI Reference In"=w6218, "error in"=w6216, "Green interlace ON count"="GI Frequency, ON count", "Green interlace OFF count"="GI Frequency, OFF count", "Green interlace ON count 2"="GI Frequency, ON count", "Green interlace OFF count 2"="GI Frequency, OFF count", "Green FB Count"="Green FB Count") -> ("error out"=w6217:errorcluster)  [unwired: 1 out]
      }
      event "Number of F/B Scans (AOD)", "Scan Speed (nm/s)", "Scan BD", "Initial delta (MHz)", "Step Size (nm)", "Scan Range (nm)": Value Change {
        w6397 = 123.0  # AOM cal (nm/MHz)
        n1411 = event-data() -> ()  [unwired: 7 out]
        n1412 = local read "BD 1 Frequency 1 (MHz)"() -> (w6380:dbl)
        n1413 = local read "AOM X Cal (nm/MHz)"() -> (w6372:dbl)
        n1414 = local read "X RF Frequency Limits (MHz)"() -> (w6384:T17)
        n1415 = local read "Y RF Frequency Limits (MHz)"() -> (w6381:T17)
        n1416 = local read "BD 2 Frequency 1 (MHz)"() -> (w6386:dbl)
        n1417 = Negate(x="Scan Range (nm)") -> (-x=w6350:dbl)
        n1418 = Divide(x=w6350, y=w6372) -> (x/y=w6354:dbl)
        n1419 = Select(t=w6384, s="Scan BD", f=w6381) -> (s? t:f=w6383:T17)
        n1420 = Select(t=w6380, s="Scan BD", f=w6386) -> (s? t:f=w6385:dbl)
        n1421 = Unbundle By Name(w6383) -> ("Maximum"=w6392:dbl, "Minimum"=w6391:dbl)
        n1422 = Add(x=w6354, y=w6385) -> (x+y=w6389:dbl)
        n1423 = Divide(x=w6350, y="Step Size (nm)") -> (x/y=w6369:dbl)
        n1424 = Divide(x="Step Size (nm)", y=w6372) -> (x/y=w6378:dbl)
        n1425 = Absolute Value(x=w6369) -> (abs(x)=w6353:dbl)
        n1426 = Sign(1:w6350) -> (0:w6351:dbl)
        n1427 = In Range and Coerce(upper limit=w6392, x=w6389, lower limit=w6391) -> (coerced(x)=w6388:dbl, In Range?=w6390:bool)
        n1428 = To Unsigned Quad Integer(1:w6353) -> (0:w6368:u64)
        "Scan steps (AOD)" <- w6368
        n1429 = call "IR AOM freq to word.vi"("Frequency In (MHz)"=w6378) -> ("Frequency Word Out (double)"=w6375:dbl)
        n1430 = Multiply(x=w6351, y=w6375) -> (x*y=w6352:dbl)
        n1431 = Subtract(x=w6389, y=w6388) -> (x-y=w6387:dbl)
        n1432 = To Quad Integer(1:w6352) -> (0:w6374:i64)
        "Incr. int (AOD)" <- w6374
        n1433 = Subtract(x=w6354, y=w6387) -> (x-y=w6373:dbl)
        "Scan Range (MHz)" <- w6373
        n1434 = Select(t=w6354, s=w6390, f=w6373) -> (s? t:f=w6393:dbl)
        n1435 = Multiply(x=w6373, y=w6372) -> (x*y=w6371:dbl)
        n1436 = Decrement(x=w6368) -> (x-1=w6421:u64)
        n1437 = Negate(x=w6371) -> (-x=w6367:dbl)
        n1438 = local write "Scan Range (nm)"(w6367) -> ()
        n1439 = Divide(x=w6393, y=w6421) -> (x/y=w6377:dbl)
        "Scan Increment (MHz)" <- w6377
        n1440 = call "IR AOM freq to word.vi"("Frequency In (MHz)"=w6377) -> ("Frequency Word Out (double)"=w6376:dbl)
        n1441 = Divide(x="Step Size (nm)", y="Scan Speed (nm/s)") -> (x/y=w6364:dbl)
        n1442 = To Quad Integer(1:w6376) -> ()  [unwired: 1 out]
        n1443 = local read "Number Interlace Sets"() -> (w6348:u8)
        n1444 = local read "AI Count (ticks)"() -> (w6349:u32)
        n1445 = local read "Total Counts (ticks)"() -> (w6347:u32)
        n1446 = local read "# Samples/trap"() -> (w6379:u32)
        n1447 = Multiply(x=w6349, y=w6348) -> (x*y=w6346:u32)
        n1448 = Divide(x=w6347, y=w6346) -> (x/y=w6345:dbl)
        n1449 = Select(t=w6380, s="Scan BD", f=w6386) -> (s? t:f=w6418:dbl)
        "Initial freq. (MHz)" <- w6418
        n1450 = Add(x=w6393, y=w6418) -> (x+y=→"Final freq. (MHz)":dbl)
        n1451 = Divide(x=w6347, y=40000000.0) -> (x/y=w6363:dbl)
        n1452 = Divide(x=w6364, y=w6363) -> (x/y=w6362:dbl)
        n1453 = To Unsigned Quad Integer(1:w6362) -> (0:w6337:u64)
        n1454 = Quotient & Remainder(x=w6337, y=u64 2) -> (x-y*floor(x/y)=w6341:u64)  [unwired: 1 out]
        n1455 = Equal?(x=w6341, y=u64 0) -> (x = y?=w6339:bool)
        n1456 = Decrement(x=w6337) -> (x-1=w6338:u64)
        n1457 = Select(t=w6337, s=w6339, f=w6338) -> (s? t:f=w6336:u64)
        "Cycles/step (AOD)" <- w6336
        n1458 = xnode "Read/Write Control"("FPGA VI Reference In"=w6429, "error in"=w6428, "Scan steps"=w6368, "Number of scans"="Number of F/B Scans (AOD)", "Cycles per step"=w6336, "Scan freq.  increment"=w6374, "Scan BD"="Scan BD") -> ("error out"=w6427:errorcluster)  [unwired: 1 out]
        n1459 = Multiply(x=w6368, y=w6336) -> (x*y=w6422:u64)
        n1460 = Multiply(x=w6422, y=u64 2) -> (x*y=w6344:u64)
        n1461 = Multiply(x=w6345, y=w6344) -> (x*y=w6343:dbl)
        "Data points/scan (f/b)" <- w6343
        n1462 = Multiply(x=w6343, y="Number of F/B Scans (AOD)") -> (x*y=w6425:dbl)
        "Data points/scans" <- w6425
        n1463 = Divide(x=w6425, y=w6379) -> (x/y=→"N sets should be saved":dbl)
        n1464 = Multiply(x=w6422, y=w6363) -> (x*y=w6361:dbl)
        "Time/Scan (s) (AOD)" <- w6361
        n1465 = Select(t=w6393, s="Scan BD", f=0.0) -> (s? t:f=w6419:dbl)
        n1466 = Select(t=0.0, s="Scan BD", f=w6393) -> (s? t:f=w6415:dbl)
        n1467 = local read "BD 2 Frequency 2 (MHz)"() -> (w6411:dbl)
        n1468 = local read "BD 1 Frequency 2 (MHz)"() -> (w6414:dbl)
        n1469 = Add(x=w6415, y=w6386) -> (x+y=w6412:dbl)
        n1470 = Add(x=w6380, y=w6419) -> (x+y=w6413:dbl)
        n1471 = Multiply(x=w6361, y=2.0) -> (x*y=w6360:dbl)
        n1472 = Multiply(x=w6360, y="Number of F/B Scans (AOD)") -> (x*y=w6357:dbl)
        n1473 = Divide(x=w6357, y=60.0) -> (x/y=→"Time to Finish All (min)":dbl)
        n1474 = Add(x="Trap 2 Bead Size (nm)", y="Trap 1 Bead Size (nm)") -> (x+y=w6401:dbl)
        n1475 = Divide(x=w6401, y=2.0) -> (x/y=w6395:dbl)
        n1476 = local read "Initial delta (MHz)"() -> (w6398:dbl)
        n1477 = Subtract(x=w6412, y=w6411) -> (x-y=w6409:dbl)
        n1478 = Subtract(x=w6413, y=w6414) -> (x-y=w6410:dbl)
        n1479 = Square(x=w6409) -> (x^2=w6408:dbl)
        n1480 = Square(x=w6410) -> (x^2=w6407:dbl)
        n1481 = Add(x=w6407, y=w6408) -> (x+y=w6406:dbl)
        n1482 = Square Root(x=w6406) -> (sqrt(x)=w6405:dbl)
        "Final delta (MHz)" <- w6405
        n1483 = Multiply(x=w6397, y=w6405) -> (x*y=w6404:dbl)
        n1484 = Multiply(x=w6398, y=w6397) -> (x*y=w6396:dbl)
        n1485 = Subtract(x=w6396, y=w6395) -> (x-y=→"Initial sep (nm)":dbl)
        n1486 = Subtract(x=w6404, y=w6395) -> (x-y=→"Final sep (nm)":dbl)
      }
      event "Freq or Amp switch first", "Swap F1 and F2", "Freq switch delay", "Amp switch delay": Value Change {
        n1487 = event-data() -> ()  [unwired: 7 out]
        n1488 = local read "Freq or Amp switch first"() -> (w6566:bool)
        n1489 = local read "Amp switch delay"() -> (w6567:u16)
        n1490 = local read "Freq switch delay"() -> (w6569:u16)
        n1491 = local read "Swap F1 and F2"() -> (w6568:bool)
        n1492 = xnode "Read/Write Control"("FPGA VI Reference In"=w6572, "error in"=w6571, "Freq switch delay"=w6569, "Swap F1 and F2"=w6568, "Amp switch delay"=w6567, "Freq or Amp switch first"=w6566) -> ("error out"=w6570:errorcluster)  [unwired: 1 out]
      }
      event "Scan steps (MCL)", "Number of scans (MCL)", "Scan Range (V)\n(of steps)", "2D or 1D Scan", "N APD Samp/step", "Fast Scan Dir", "Continuous MCL Scanning", "Scan lines (y)": Value Change {
        w6673 = 32767.0 ("y")
        n1493 = event-data() -> ()  [unwired: 7 out]
        n1494 = Select(t="Scan lines (y)", s="2D or 1D Scan", f="Number of scans (MCL)") -> (s? t:f=w6678:u64)
        n1495 = Decrement(x="Scan steps (MCL)") -> (x-1=w6694:u64)
        n1496 = Divide(x="Scan Range (V)\n(of steps)", y=w6694) -> (x/y=w6693:dbl)
        "Desired Scan Incr (V)" <- w6693
        n1497 = local read "APD Integration Time (s)"() -> (w6686:dbl)
        n1498 = Multiply(x=w6693, y=w6673) -> (x*y=w6702:dbl)
        n1499 = Divide(x=w6702, y=10.0) -> (x/y=w6692:dbl)
        "Desired incr (int)" <- w6692
        n1500 = local read "Update Count (MCL)"() -> (w6698:u32)
        n1501 = Round Toward -Infinity(1:w6692) -> (0:w6701:dbl)
        n1502 = To Word Integer(number=w6701) -> (16bit integer=w6676:i16)
        "Actual Incr. int (MCL)" <- w6676
        n1503 = Multiply(x=w6686, y=40000000.0) -> (x*y=w6699:dbl)
        n1504 = Divide(x=w6699, y=w6698) -> (x/y=w6697:dbl)
        n1505 = Multiply(x=i16 10, y=w6676) -> (x*y=w6674:i16)
        n1506 = Multiply(x="N APD Samp/step", y=w6697) -> (x*y=w6696:dbl)
        "Cycles/step (MCL)" <- w6696
        n1507 = Divide(x=w6674, y=w6673) -> (x/y=→"Actual MCL Inc (V)":dbl)
        n1508 = Multiply(x="N APD Samp/step", y="Scan steps (MCL)") -> (x*y=w6688:dbl)
        n1509 = local read "APD Samples/FIFO Acq."() -> (w6685:dbl)
        n1510 = Multiply(x=w6688, y=u64 2) -> (x*y=w6687:dbl)
        "Data points/scan (f+b)" <- w6687
        n1511 = Multiply(x=w6687, y=w6678) -> (x*y=w6705:dbl)
        "Data points/scans (MCL)" <- w6705
        n1512 = Multiply(x=w6686, y=w6687) -> (x*y=w6679:dbl)
        "Time/f+b scan (s) (MCL)" <- w6679
        n1513 = Divide(x=w6705, y=w6685) -> (x/y=→"N sets should be saved (MCL)":dbl)
        n1514 = Multiply(x=w6679, y=w6678) -> (x*y=→"Total Time (s)":dbl)
        n1515 = Not(x="Fast Scan Dir") -> (.not. x?=w6683:bool)
        n1516 = xnode "Read/Write Control"("FPGA VI Reference In"=w6709, "error in"=w6708, "Scan steps (MCL)"="Scan steps (MCL)", "Number of scans (MCL)"=w6678, "Cycles per step (MCL)"=w6696, "Scan freq.  increment (MCL)"=w6676, "1D or 2D Scan?"="2D or 1D Scan", "MCL Scan Axis"=w6683, "Cont. Scan (MCL)"="Continuous MCL Scanning") -> ("error out"=w6707:errorcluster)  [unwired: 1 out]
      }
      event Key Down {
        n1517 = event-data() -> ("VKey"=w6883:T47)  [unwired: 10 out]
        n1518 = local read "z nudge increment (um)"() -> (w6882:dbl)
        n1519 = case shown="\"PageDown\"" w6883 {
          tunnel: "lateral step size (mm)" -> [w6886 w6891 w6896 w6904 _ _ _ _ _ _ _ _ _ _ _ _ _ _ _ _ _ _ _ _ _ _ _ _ _ _ _ _ _ _ _ _ _ _ _ _ _ _ _ _ _ _ _ _ _ _ _ _ _ _ _ _]
          tunnel: w6882 -> [_ _ _ _ w6907 w6914 _ _ _ _ _ _ _ _ _ _ _ _ _ _ _ _ _ _ _ _ _ _ _ _ _ _ _ _ _ _ _ _ _ _ _ _ _ _ _ _ _ _ _ _ _ _ _ _ _ _]
          frame "Up" {
            w6888 = 0.0 ("element")
            n1520 = Negate(x=w6886) -> (-x=w6885:dbl)
            n1521 = Build Array(w6888, w6885, w6888) -> (w6887:dbl[])
            n1522 = call "CONEX_FUNCTIONAL_GLOBAL.vi"("Axis"=enum16{"X", "Y", "Z", "XY", "XZ", "YZ", "XYZ"}."Y", "Position"=w6887, "Command"=T23."REL MOVE") -> ()  [unwired: 6 in, 3 out]
          }
          frame "Down" {
            w6893 = 0.0 ("element")
            n1523 = Build Array(w6893, w6891, w6893) -> (w6892:dbl[])
            n1524 = call "CONEX_FUNCTIONAL_GLOBAL.vi"("Axis"=enum16{"X", "Y", "Z", "XY", "XZ", "YZ", "XYZ"}."Y", "Position"=w6892, "Command"=T23."REL MOVE") -> ()  [unwired: 6 in, 3 out]
          }
          frame "Left" {
            w6897 = 0.0 ("element")
            n1525 = Build Array(w6896, w6897, w6897) -> (w6898:dbl[])
            n1526 = call "CONEX_FUNCTIONAL_GLOBAL.vi"("Axis"=enum16{"X", "Y", "Z", "XY", "XZ", "YZ", "XYZ"}."X", "Position"=w6898, "Command"=T23."REL MOVE") -> ()  [unwired: 6 in, 3 out]
          }
          frame "Right" {
            w6902 = 0.0 ("element")
            n1527 = Negate(x=w6904) -> (-x=w6903:dbl)
            n1528 = Build Array(w6903, w6902, w6902) -> (w6901:dbl[])
            n1529 = call "CONEX_FUNCTIONAL_GLOBAL.vi"("Axis"=enum16{"X", "Y", "Z", "XY", "XZ", "YZ", "XYZ"}."X", "Position"=w6901, "Command"=T23."REL MOVE") -> ()  [unwired: 6 in, 3 out]
          }
          frame "PageUp" {
            w6911 = 0.0 ("element")
            n1530 = Divide(x=w6907, y=1000.0) -> (x/y=w6909:dbl)
            n1531 = Build Array(w6911, w6911, w6909) -> (w6910:dbl[])
            n1532 = call "CONEX_FUNCTIONAL_GLOBAL.vi"("Axis"=enum16{"X", "Y", "Z", "XY", "XZ", "YZ", "XYZ"}."Z", "Position"=w6910, "Command"=T23."REL MOVE") -> ()  [unwired: 6 in, 3 out]
          }
          frame "PageDown" {
            w6918 = 0.0 ("element")
            n1533 = Divide(x=w6914, y=-1000.0) -> (x/y=w6916:dbl)
            n1534 = Build Array(w6918, w6918, w6916) -> (w6917:dbl[])
            n1535 = call "CONEX_FUNCTIONAL_GLOBAL.vi"("Axis"=enum16{"X", "Y", "Z", "XY", "XZ", "YZ", "XYZ"}."Z", "Position"=w6917, "Command"=T23."REL MOVE") -> ()  [unwired: 6 in, 3 out]
          }
          frame Default {
          }
          frame "Insert" {
          }
          frame "Delete" {
          }
          frame "Home" {
          }
          frame "End" {
          }
          frame "Escape" {
          }
          frame "Help" {
          }
          frame "Pause" {
          }
          frame "ScrollLock" {
          }
          frame "F1" {
          }
          frame "F2" {
          }
          frame "F3" {
          }
          frame "F4" {
          }
          frame "F5" {
          }
          frame "F6" {
          }
          frame "F7" {
          }
          frame "F8" {
          }
          frame "F9" {
          }
          frame "F10" {
          }
          frame "F11" {
          }
          frame "F12" {
          }
          frame "F13" {
          }
          frame "F14" {
          }
          frame "F15" {
          }
          frame "F16" {
          }
          frame "F17" {
          }
          frame "F18" {
          }
          frame "F19" {
          }
          frame "F20" {
          }
          frame "F21" {
          }
          frame "F22" {
          }
          frame "F23" {
          }
          frame "F24" {
          }
          frame "Play" {
          }
          frame "VolumeUp" {
          }
          frame "VolumeDown" {
          }
          frame "Mute" {
          }
          frame "Two Byte Char" {
          }
          frame "Break" {
          }
          frame "Clear" {
          }
          frame "NumLock" {
          }
          frame "Caps" {
          }
          frame "Opt" {
          }
          frame "Cmd" {
          }
          frame "Alt" {
          }
          frame "Ctrl" {
          }
          frame "Shift" {
          }
          frame "Return" {
          }
          frame "Enter" {
          }
          frame "ASCII" {
          }
        }
      }
      event "Read Cal": Value Change {
        w6922 = 1000.0 ("y")
        n1536 = event-data() -> ()  [unwired: 7 out]
        n1537 = local read "Save file name"() -> (w6947:path)
        n1538 = local write "Read Cal"(FALSE ("Read Cal")) -> ()
        n1539 = Strip Path(path=w6947) -> (stripped path=w6946:path)  [unwired: 1 out]
        n1540 = Path To String(path=w6946) -> (string=w6945:string)
        n1541 = Concatenate Strings(w6945, "\\current.cal" ("string")) -> (w6943:string)
        n1542 = String To Path(string=w6943) -> (path=w6942:path)
        n1543 = Open/Create/Replace File(file path (use dialog)=w6942, operation (0:open)=T37."open", access (0:read/write)=enum16{"read/write", "read-only", "write-only"}."read-only") -> (refnum out=w6950:refnum<file>, error out=w6936:errorcluster)  [unwired: 1 in, 3 out]
        n1544 = Deny Access(4:w6936, 7:w6950) -> (0:w6935:errorcluster, 3:w6941:refnum<file>)  [unwired: 1 out]